vi "UHR-Fleezers Control (host) - 12.7d.vi"() -> ()   [LabVIEW 2012] (continued)
            n1305 = property on="Fish for Tether" class="Bool (strict)"("Val(Sgnl)"=TRUE ("Value (Signaling)")) -> ()  [unwired: 2 in, 2 out]
          }
        }
        n1306 = local write "Cal/Data Acq. Spot"(FALSE ("Cal/Data Acq. Spot")) -> ()
      }
      event "Dump Beads": Value Change {
        n1307 = event-data() -> ()  [unwired: 1 in, 5 out]
        n1308 = flat-sequence {
          tunnel: ["Dump spot flow on?"] -> w1942
          tunnel: [w1953] -> w1943
          tunnel: w1942 -> [w1953]
          tunnel: w1946 -> [w1958]
          tunnel: w1945 -> [w1957]
          tunnel: [w1955] -> w1944
          tunnel: w1943 -> [w1955]
          tunnel: w1944 -> [w1968]
          frame #0 {
            w1947 = FALSE ("Value (Signaling)")
            n1309 = local read "Saving..."() -> (w1949:bool)
            n1310 = local write "Dump Beads"(FALSE ("Dump Beads")) -> ()
            n1311 = property on="Inject Pump 3" class="Bool (strict)"("Val(Sgnl)"=w1947) -> ()  [unwired: 2 in, 2 out]
            n1312 = property on="Inject Pump 1" class="Bool (strict)"("Val(Sgnl)"=w1947) -> ()  [unwired: 2 in, 2 out]
            n1313 = local write "Stop Saving"(w1949) -> ()
          }
          frame #1 {
            w1950 = FALSE ("Fl. Triggered...")
            n1314 = case shown="True" "Dump spot flow on?" {
              frame False {
              }
              frame True {
                n1315 = property on="Sample Channel\nFlow" class="Bool (strict)"("Val(Sgnl)"=TRUE ("Stage Moving")) -> ()  [unwired: 2 in, 2 out]
              }
            }
            n1316 = local write "Fl. Triggered..."(w1950) -> ()
            n1317 = local write "Tether"(w1950) -> ()
            n1318 = property on="Green Laser ON" class="Bool (strict)"("Val(Sgnl)"=w1950) -> ()  [unwired: 2 in, 2 out]
            n1319 = property on="Trap Pos. FB ON" class="Bool (strict)"("Val(Sgnl)"=w1950) -> ()  [unwired: 2 in, 2 out]
            n1320 = property on="Trap Trig. Fl." class="Bool (strict)"("Val(Sgnl)"=w1950) -> ()  [unwired: 2 in, 2 out]
            n1321 = property on="Fl. Triggered..." class="Bool (strict)"("Val(Sgnl)"=w1950) -> ()  [unwired: 2 in, 2 out]
            n1322 = property on="Dip for Protein" class="Bool (strict)"("Val(Sgnl)"=w1950) -> ()  [unwired: 2 in, 2 out]
            n1323 = property on="Pause dwell" class="Bool (strict)"("Val(Sgnl)"=w1950) -> ()  [unwired: 2 in, 2 out]
          }
          frame #2 {
            n1324 = property on="Trap Pos. FB Offset Factor" class="DigNum (strict)"("Val(Sgnl)"=i64 0 ("Value (Signaling)")) -> ()  [unwired: 2 in, 2 out]
          }
          frame #3 {
            n1325 = local read "Saved Stage Positions"() -> (w1959:dbl[][])
            n1326 = local write "Stage Moving"(TRUE ("Stage Moving")) -> ()
            n1327 = Array Subset(array=w1959, index (row)=3 ("index"), length (row)=1 ("length"), index (col)=1 ("index"), length (col)=3 ("length")) -> (w1964:dbl[][])
            n1328 = Reshape Array(w1964, 3 ("dimension size")) -> (w1962:dbl[])
            n1329 = Array To Cluster(array=w1962) -> (cluster=w1961:cluster{"[0]":dbl, "[1]":dbl, "[2]":dbl})
            n1330 = call "Set Stage Position.vi"("Position"=w1961, "error in"=w1957, "VISA resource name in"=w1958) -> ()  [unwired: 3 out]
          }
          frame #4 {
            w1969 = FALSE ("Value (Signaling)")
            n1331 = case shown="True" w1968 {
              frame False {
              }
              frame True {
                n1332 = property on="Sample Channel\nFlow" class="Bool (strict)"("Val(Sgnl)"=FALSE ("Stage Moving")) -> ()  [unwired: 2 in, 2 out]
              }
            }
            n1333 = property on="Trap 1 (ON/OFF)" class="Bool (strict)"("Val(Sgnl)"=w1969) -> ()  [unwired: 2 in, 2 out]
            n1334 = property on="Trap 2 (ON/OFF)" class="Bool (strict)"("Val(Sgnl)"=w1969) -> ()  [unwired: 2 in, 2 out]
            n1335 = call <vilib>:"Beep.vi"() -> ()  [unwired: 3 in, 9 out]
          }
          frame #5 {
            n1336 = property on="Move Cap. 2 (ADig Top)" class="Bool (strict)"("Val(Sgnl)"=TRUE ("Value (Signaling)")) -> ()  [unwired: 2 in, 2 out]
            n1337 = property on="Tab Control" class="TabCtl (strict)"("Val(Sgnl)"=T31."Status" ("Value (Signaling)")) -> ()  [unwired: 2 in, 2 out]
          }
        }
      }
      event "Dip for Protein": Value Change {
        n1338 = event-data() -> ()  [unwired: 1 in, 5 out]
        n1339 = case shown="True" "Dip for Protein" {
          tunnel: w1975 -> [_ w1977]
          tunnel: w1974 -> [_ w1976]
          frame False {
          }
          frame True {
            n1340 = while {
              tunnel: w1977 -> [w1988]
              tunnel: w1976 -> [w1987]
              i -> [w1982]
              stop <- w1984 stop-if-true
              n1341 = Increment(x=w1982) -> (x+1=→"Dip #":i32)
              n1342 = flat-sequence {
                tunnel: w1987 -> [w1999]
                tunnel: w1988 -> [w2000]
                tunnel: [w2000] -> w1992
                tunnel: [w1999] -> w1991
                tunnel: [w1993] -> w1978
                tunnel: [w2005] -> w1986
                tunnel: [w2006] -> w1985
                tunnel: w1992 -> [w2007]
                tunnel: w1991 -> [w2008]
                tunnel: [w2003] -> w1979
                tunnel: w1978 -> [w2003]
                tunnel: [w2016] -> w1990
                tunnel: w1986 -> [w2016]
                tunnel: [w2015] -> w1989
                tunnel: w1985 -> [w2015]
                tunnel: [w2012] -> w1983
                tunnel: [w2011] -> w1980
                tunnel: w1979 -> [w2011]
                tunnel: w1989 -> [w2036]
                tunnel: w1990 -> [w2037]
                tunnel: w1983 -> [w2038]
                tunnel: w1980 -> [w2035]
                tunnel: [w2094] -> w1984
                frame #0 {
                  n1343 = local read "Trap Pos. FB ON"() -> (w1993:bool)
                  n1344 = Compound Arithmetic op=AND("Flow ON\nduring dip?", "FB OFF when \nflow ON", w1993) -> (w1994:bool)
                  n1345 = case shown="True" "Move trap \nbefore dip move?" {
                    frame False {
                    }
                    frame True {
                      n1346 = property on="Trap Delta (MHz)" class="DigNum (strict)"("Val(Sgnl)"="Dipping Delta (MHz)") -> ()  [unwired: 2 in, 2 out]
                    }
                  }
                  n1347 = property on="Green Laser ON" class="Bool (strict)"("Val(Sgnl)"="Green ON\nbefore dip?") -> ()  [unwired: 2 in, 2 out]
                  n1348 = property on="Sample Channel\nFlow" class="Bool (strict)"("Val(Sgnl)"="Flow ON\nduring dip?") -> ()  [unwired: 2 in, 2 out]
                  n1349 = case shown="True" w1994 {
                    frame False {
                    }
                    frame True {
                      n1350 = property on="Trap Pos. FB ON" class="Bool (strict)"("Val(Sgnl)"=FALSE ("Value (Signaling)")) -> ()  [unwired: 2 in, 2 out]
                    }
                  }
                }
                frame #1 {
                  n1351 = local read "Saved Stage Positions"() -> (w2010:dbl[][])
                  n1352 = local write "Cancel dwell"(FALSE ("Cancel dwell")) -> ()
                  n1353 = call "move to saved stage position.vi"("error in"=w2008, "Stage VISA resource name in"=w2007, "Position"="Dip Stage \nPosition", "Saved Stage Positions"=w2010) -> ("VISA resource name out"=w2005:refnum<visa-resource-name>, "error out"=w2006:errorcluster)
                }
                frame #2 {
                  n1354 = node-c288() -> (w2014:T23)  [unwired: 4 in]
                  n1355 = timed-loop {
                    timing: w2014 -> [_]
                    timing-out: [_] -> w2013
                    tunnel: [w2020] -> w2012
                    i -> [w2017]
                    stop <- w2021 stop-if-true
                    n1356 = node-c288() -> ()  [unwired: 1 in, 1 out]
                    n1357 = Greater Or Equal?(x=w2017, y="Dip Duration (s)") -> (x >= y?=w2029:bool)
                    n1358 = local read "Dip for Protein"() -> (w2022:bool)
                    n1359 = local read "Dump Beads"() -> (w2019:bool)
                    n1360 = local read "Cancel dwell"() -> (w2028:bool)
                    n1361 = local read "Pause dwell"() -> (w2025:bool)
                    n1362 = Not(x=w2022) -> (.not. x?=w2027:bool)
                    n1363 = Compound Arithmetic op=OR(w2028, w2029, w2027) -> (w2026:bool)
                    n1364 = Select(t=FALSE, s=w2025, f=w2026) -> (s? t:f=w2023:bool)
                    n1365 = Not(x=w2019) -> (.not. x?=w2018:bool)
                    n1366 = node-c288() -> ()  [unwired: 1 in, 1 out]
                    n1367 = And(x=w2022, y=w2018) -> (x .and. y?=w2020:bool)
                    n1368 = Or(x=w2023, y=w2019) -> (x .or. y?=w2021:bool)
                    "Dip Time (s)" <- w2017
                  }
                  n1369 = node-c288(w2013) -> ()  [unwired: 1 out]
                }
                frame #3 {
                  n1370 = case shown="True" w2038 {
                    tunnel: w2037 -> [_ w2043]
                    tunnel: w2036 -> [_ w2042]
                    tunnel: w2035 -> [_ w2039]
                    frame False {
                    }
                    frame True {
                      n1371 = flat-sequence {
                        tunnel: w2042 -> [w2047]
                        tunnel: w2043 -> [w2048]
                        tunnel: [w2048] -> w2041
                        tunnel: [w2047] -> w2040
                        tunnel: w2039 -> [w2044]
                        tunnel: w2041 -> [w2058]
                        tunnel: w2040 -> [w2057]
                        tunnel: w2039 -> [w2066]
                        frame #0 {
                          n1372 = local read "Sample Channel\nFlow"() -> (w2046:bool)
                          n1373 = case shown="True" w2046 {
                            tunnel: "Flow ON \nduring return\nfrom dip?" -> [w2049 w2052]
                            tunnel: w2044 -> [_ w2051]
                            frame False {
                              n1374 = case shown="True" w2049 {
                                frame False {
                                }
                                frame True {
                                n1375 = property on="Sample Channel\nFlow" class="Bool (strict)"("Val(Sgnl)"=TRUE ("Value (Signaling)")) -> ()  [unwired: 2 in, 2 out]
                                }
                              }
                            }
                            frame True {
                              n1376 = case shown="False" w2052 {
                                tunnel: w2051 -> [w2053 _]
                                frame False {
                                n1377 = property on="Trap Pos. FB ON" class="Bool (strict)"("Val(Sgnl)"=w2053) -> ()  [unwired: 2 in, 2 out]
                                n1378 = property on="Sample Channel\nFlow" class="Bool (strict)"("Val(Sgnl)"=FALSE ("Value (Signaling)")) -> ()  [unwired: 2 in, 2 out]
                                }
                                frame True {
                                }
                              }
                            }
                          }
                        }
                        frame #1 {
                          # "For turning on green laser before stage reaches lower spot"
                          n1379 = case shown="True" "Green ON\nafter start\nreturn?" {
                            frame False {
                            }
                            frame True {
                              n1380 = flat-sequence {
                                frame #0 {
                                n1381 = Multiply(x="Green delay after \nstart return (s)", y=1000.0) -> (x*y=w2063:dbl)
                                n1382 = Wait (ms)(milliseconds to wait=w2063) -> ()  [unwired: 1 out]
                                }
                                frame #1 {
                                n1383 = property on="Green Laser ON" class="Bool (strict)"("Val(Sgnl)"=TRUE ("Value (Signaling)")) -> ()  [unwired: 2 in, 2 out]
                                }
                              }
                            }
                          }
                          n1384 = local read "Saved Stage Positions"() -> (w2061:dbl[][])
                          n1385 = local write "Cancel dwell"(FALSE ("Cancel dwell")) -> ()
                          n1386 = call "move to saved stage position.vi"("error in"=w2057, "Stage VISA resource name in"=w2058, "Position"="Return Stage \nPosition", "Saved Stage Positions"=w2061) -> ("error out"=w2059:errorcluster)  [unwired: 1 out]
                          n1387 = local write "Stage Control Serial Error"(w2059) -> ()
                        }
                        frame #2 {
                          n1388 = property on="Trap Pos. FB ON" class="Bool (strict)"("Val(Sgnl)"=w2066) -> ()  [unwired: 2 in, 2 out]
                          n1389 = case shown="True" "Green ON \nafter return?" {
                            frame False {
                            }
                            frame True {
                              n1390 = property on="Green Laser ON" class="Bool (strict)"("Val(Sgnl)"=TRUE ("Value (Signaling)")) -> ()  [unwired: 2 in, 2 out]
                            }
                          }
                          n1391 = case shown="True" "Move trap after return?" {
                            frame False {
                            }
                            frame True {
                              n1392 = property on="Trap Delta (MHz)" class="DigNum (strict)"("Val(Sgnl)"="Dip Trap Delta 2 (MHz)") -> ()  [unwired: 2 in, 2 out]
                            }
                          }
                          n1393 = case shown="True" "Save data after return?" {
                            frame False {
                            }
                            frame True {
                              n1394 = property on="Start Saving" class="Bool (strict)"("Val(Sgnl)"=TRUE ("Value (Signaling)")) -> ()  [unwired: 2 in, 2 out]
                            }
                          }
                          n1395 = property on="Sample Channel\nFlow" class="Bool (strict)"("Val(Sgnl)"="Flow ON\nduring daq?") -> ()  [unwired: 2 in, 2 out]
                        }
                        frame #3 {
                          n1396 = node-c288() -> (w2075:T23)  [unwired: 4 in]
                          n1397 = timed-loop {
                            timing: w2075 -> [_]
                            timing-out: [_] -> w2074
                            i -> [w2076]
                            stop <- w2078 stop-if-true
                            n1398 = node-c288() -> ()  [unwired: 1 in, 1 out]
                            n1399 = local read "Dump Beads"() -> (w2077:bool)
                            n1400 = Greater Or Equal?(x=w2076, y="Dwell Duration (s)") -> (x >= y?=w2083:bool)
                            n1401 = local read "Dip for Protein"() -> (w2080:bool)
                            n1402 = Not(x=w2080) -> (.not. x?=w2079:bool)
                            n1403 = Compound Arithmetic op=OR(w2083, "Cancel dwell", w2079) -> (w2082:bool)
                            n1404 = node-c288() -> ()  [unwired: 1 in, 1 out]
                            n1405 = Select(t=FALSE, s="Pause dwell", f=w2082) -> (s? t:f=w2085:bool)
                            n1406 = Or(x=w2085, y=w2077) -> (x .or. y?=w2078:bool)
                            "Dwell Time (s)" <- w2076
                          }
                          n1407 = node-c288(w2074) -> ()  [unwired: 1 out]
                        }
                      }
                    }
                  }
                }
                frame #4 {
                  n1408 = local read "Dip for Protein"() -> (w2095:bool)
                  n1409 = local read "Dump Beads"() -> (w2092:bool)
                  n1410 = local write "Cancel dwell"(FALSE ("Cancel dwell")) -> ()
                  n1411 = Not(x=w2095) -> (.not. x?=w2096:bool)
                  n1412 = Not(x="Cont. Repeat Dipping?") -> (.not. x?=w2098:bool)
                  n1413 = Compound Arithmetic op=OR(w2096, w2098, w2092) -> (w2094:bool)
                }
              }
            }
          }
        }
      }
      event "Profile": Value Change {
        n1414 = event-data() -> ()  [unwired: 1 in, 5 out]
        n1415 = flat-sequence {
          tunnel: w2107 -> [w2110]
          tunnel: w2106 -> [w2118]
          tunnel: [w2112] -> w2105
          tunnel: [w2111] -> w2104
          tunnel: [w2109] -> w2102
          tunnel: [w2108] -> w2099
          tunnel: w2105 -> [w2125]
          tunnel: w2104 -> [w2124]
          tunnel: [w2122] -> w2103
          tunnel: w2102 -> [w2123]
          tunnel: [w2121] -> w2101
          tunnel: [w2120] -> w2100
          tunnel: w2099 -> [w2120]
          tunnel: w2103 -> [w2129]
          tunnel: w2101 -> [w2128]
          tunnel: w2100 -> [w2127]
          frame #0 {
            n1416 = call "Read Stage Position.vi"("error in"=w2118, "VISA resource name in"=w2110) -> ("Current Position"=w2108:cluster{dbl, dbl, dbl}, "error out"=w2111:errorcluster, "VISA resource name out"=w2109:refnum<visa-resource-name>)  [unwired: 1 out]
            "Current Position" <- w2108
            n1417 = local write "Stage Control Serial Error"(w2111) -> ()
            n1418 = Unbundle(w2108) -> (w2115:dbl, w2117:dbl, w2113:dbl)
            n1419 = Add(x=w2117, y="Y change (mm)") -> (x+y=w2114:dbl)
            n1420 = Bundle(w2115, w2114, w2113) -> (w2112:cluster{dbl, dbl, dbl})  [unwired: 1 in]
          }
          frame #1 {
            # "move to new position and start saving"
            n1421 = local write "Stage Moving"(TRUE ("Stage Moving")) -> ()
            n1422 = local write "Start Saving"(TRUE ("Start Saving")) -> ()
            n1423 = call "Set Stage Position.vi"("Position"=w2125, "error in"=w2124, "VISA resource name in"=w2123) -> ("error out"=w2121:errorcluster, "VISA resource name out"=w2122:refnum<visa-resource-name>)  [unwired: 1 out]
          }
          frame #2 {
            # "go back to start"
            n1424 = call "Set Stage Position.vi"("Position"=w2127, "error in"=w2128, "VISA resource name in"=w2129) -> ()  [unwired: 3 out]
          }
          frame #3 {
            # "stop saving"
            n1425 = local write "Stop Saving"(TRUE ("Stop Saving")) -> ()
            n1426 = local write "Stage Moving"(FALSE ("Stage Moving")) -> ()
          }
        }
      }
      event "Move to Position 1", "Move to Position 2", "Move to Position 3", "Move to Position 4", "Move to Position 5", "Lower Ch. Cap.": Value Change {
        n1427 = event-data() -> ()  [unwired: 1 in, 5 out]
        n1428 = Or(x="Move to Position 5", y="Lower Ch. Cap.") -> (x .or. y?=w2135:bool)
        n1429 = Build Array("Move to Position 1", "Move to Position 2", "Move to Position 3", "Move to Position 4", w2135) -> (w2138:bool[])
        n1430 = Boolean Array To Number(Boolean array=w2138) -> (number=w2137:u32)
        n1431 = Logarithm Base 2(1:w2137) -> (0:w2136:dbl)
        n1432 = flat-sequence {
          tunnel: w2136 -> [w2147]
          tunnel: w2133 -> [w2145]
          tunnel: w2132 -> [w2144]
          frame #0 {
            n1433 = local read "Saved Stage Positions"() -> (w2155:dbl[][])
            n1434 = Array Subset(array=w2155, index (row)=w2147, length (row)=1 ("length"), index (col)=1 ("index"), length (col)=3 ("length")) -> (w2152:dbl[][])
            n1435 = Reshape Array(w2152, 3 ("dimension size")) -> (w2150:dbl[])
            n1436 = Array To Cluster(array=w2150) -> (cluster=w2149:cluster{"[0]":dbl, "[1]":dbl, "[2]":dbl})
            n1437 = call "Set Stage Position.vi"("Position"=w2149, "error in"=w2144, "VISA resource name in"=w2145) -> ("error out"=w2148:errorcluster)  [unwired: 2 out]
            n1438 = local write "Stage Moving"(TRUE ("Stage Moving")) -> ()
            n1439 = local write "Stage Control Serial Error"(w2148) -> ()
          }
          frame #1 {
            n1440 = local write "Stage Moving"(FALSE ("Stage Moving")) -> ()
            n1441 = call <vilib>:"Beep.vi"() -> ()  [unwired: 3 in, 9 out]
          }
        }
      }
      event "Got ADig bead": Value Change {
        n1442 = event-data() -> ()  [unwired: 1 in, 5 out]
        n1443 = flat-sequence {
          frame #0 {
            n1444 = local read "Cap 1 Samp Flow ON"() -> (w2159:bool)
            n1445 = case shown="True" w2159 {
              frame False {
              }
              frame True {
                n1446 = property on="Sample Channel\nFlow" class="Bool (strict)"("Val(Sgnl)"=TRUE ("Value (Signaling)")) -> ()  [unwired: 2 in, 2 out]
              }
            }
          }
          frame #1 {
            n1447 = property on="Inject Pump 3" class="Bool (strict)"("Val(Sgnl)"=FALSE ("Value (Signaling)")) -> ()  [unwired: 2 in, 2 out]
          }
          frame #2 {
            n1448 = property on="Move Cap. 1 (DNA Bottom)" class="Bool (strict)"("Val(Sgnl)"=TRUE ("Value (Signaling)")) -> ()  [unwired: 2 in, 2 out]
          }
        }
      }
      event "Force FB Data\nScript": Value Change {
        n1449 = event-data() -> ()  [unwired: 1 in, 5 out]
        n1450 = flat-sequence {
          tunnel: w2168 -> [w2172]
          tunnel: w2169 -> [w2173]
          tunnel: [w2173] -> w2164
          tunnel: [w2172] -> w2163
          tunnel: w2164 -> [w2176]
          tunnel: w2163 -> [w2175]
          tunnel: ["Trap Trig Fl."] -> w2165
          tunnel: [w2201] -> w2166
          tunnel: w2165 -> [w2201]
          tunnel: [w2205] -> w2167
          tunnel: w2166 -> [w2205]
          tunnel: w2167 -> [w2207]
          frame #0 {
            n1451 = property on="Trap Delta (MHz)" class="DigNum (strict)"("Val(Sgnl)"="Trap Delta Before Moving") -> ()  [unwired: 2 in, 2 out]
          }
          frame #1 {
            n1452 = local read "Saved Stage Positions"() -> (w2178:dbl[][])
            n1453 = local write "FB Trap Pos Offset"(0.0 ("FB Trap Pos Offset")) -> ()
            n1454 = property on="Trap Pos. FB Offset Factor" class="DigNum (strict)"("Val(Sgnl)"=i64 0 ("Value (Signaling)")) -> ()  [unwired: 2 in, 2 out]
            n1455 = local write "Stage Moving"(TRUE ("Stage Moving")) -> ()
            n1456 = call "move to saved stage position.vi"("error in"=w2175, "Stage VISA resource name in"=w2176, "Position"="Stage Position To Establish FB", "Saved Stage Positions"=w2178) -> ("error out"=w2174:errorcluster)  [unwired: 1 out]
            n1457 = local write "Stage Control Serial Error"(w2174) -> ()
          }
          frame #2 {
            n1458 = call <vilib>:"Beep.vi"() -> ()  [unwired: 3 in, 9 out]
            n1459 = Multiply(x="Wait (s)", y=u32 1000 ("milliseconds to wait")) -> (x*y=w2185:u32)
            n1460 = property on="Trap Delta (MHz)" class="DigNum (strict)"("Val(Sgnl)"="Starting \nTrap Delta (MHz)") -> ()  [unwired: 2 in, 2 out]
            n1461 = local write "Stage Moving"(FALSE ("Stage Moving")) -> ()
            n1462 = Wait (ms)(milliseconds to wait=w2185) -> ()  [unwired: 1 out]
            n1463 = property on="Tab Control 2" class="TabCtl (strict)"("Val(Sgnl)"=T6."Feedback on Trap Position" ("Value (Signaling)")) -> ()  [unwired: 2 in, 2 out]
            n1464 = property on="Tab Control" class="TabCtl (strict)"("Val(Sgnl)"=T32."Trap Control (RF)" ("Value (Signaling)")) -> ()  [unwired: 2 in, 2 out]
          }
          frame #3 {
            n1465 = property on="Set Reading to\nSetpoint" class="Bool (strict)"("Val(Sgnl)"=TRUE ("Value (Signaling)")) -> ()  [unwired: 2 in, 2 out]
            n1466 = Wait (ms)(milliseconds to wait=u32 500) -> ()  [unwired: 1 out]
          }
          frame #4 {
            n1467 = property on="Trap Pos. FB ON" class="Bool (strict)"("Val(Sgnl)"=TRUE ("Value (Signaling)")) -> ()  [unwired: 2 in, 2 out]
            n1468 = Wait (ms)(milliseconds to wait=u32 250) -> ()  [unwired: 1 out]
          }
          frame #5 {
            n1469 = case shown="False" "Trap Trig Fl." {
              frame False {
                n1470 = case shown="True" "Green ON after FB ON?" {
                  selector: "Green ON after FB ON?" -> [_ w2200]
                  frame False {
                  }
                  frame True {
                    n1471 = property on="Green Laser ON" class="Bool (strict)"("Val(Sgnl)"=w2200) -> ()  [unwired: 2 in, 2 out]
                  }
                }
              }
              frame True {
              }
            }
            n1472 = case shown="True" "Remove Action Offset" {
              tunnel: TRUE ("Value (Signaling)") -> [w2197 w2198]
              frame False {
                n1473 = property on="Remove Unwinding Offset" class="Bool (strict)"("Val(Sgnl)"=w2197) -> ()  [unwired: 2 in, 2 out]
              }
              frame True {
                n1474 = property on="Remove Action Offset" class="Bool (strict)"("Val(Sgnl)"=w2198) -> ()  [unwired: 2 in, 2 out]
              }
            }
            n1475 = Wait (ms)(milliseconds to wait=u32 250) -> ()  [unwired: 1 out]
          }
          frame #6 {
            n1476 = property on="Start Saving" class="Bool (strict)"("Val(Sgnl)"=TRUE ("Value (Signaling)")) -> ()  [unwired: 2 in, 2 out]
            n1477 = Wait (ms)(milliseconds to wait=u32 5000) -> ()  [unwired: 1 out]
          }
          frame #7 {
            w2204 = TRUE ("Value (Signaling)")
            n1478 = property on="Rem fb disp offset" class="Bool (strict)"("Val(Sgnl)"=w2204) -> ()  [unwired: 2 in, 2 out]
            n1479 = property on="Remove Offset" class="Bool (strict)"("Val(Sgnl)"=w2204) -> ()  [unwired: 2 in, 2 out]
            n1480 = Wait (ms)(milliseconds to wait=u32 100) -> ()  [unwired: 1 out]
          }
          frame #8 {
            n1481 = case shown="True" w2207 {
              frame False {
              }
              frame True {
                n1482 = local write "Trap Trig. Fl."(TRUE ("Value (Signaling)")) -> ()
              }
            }
          }
          frame #9 {
            n1483 = case shown="True" "Start dipping after?" {
              frame False {
              }
              frame True {
                n1484 = flat-sequence {
                  frame #0 {
                    n1485 = Multiply(x="Delay before dipping (s)", y=1000.0) -> (x*y=w2211:dbl)
                    n1486 = Wait (ms)(milliseconds to wait=w2211) -> ()  [unwired: 1 out]
                  }
                  frame #1 {
                    n1487 = property on="Dip for Protein" class="Bool (strict)"("Val(Sgnl)"=TRUE ("Value (Signaling)")) -> ()  [unwired: 2 in, 2 out]
                    n1488 = local write "Scripts"(T1."Dipping" ("Scripts")) -> ()
                  }
                }
              }
            }
          }
        }
      }
      event "Fixed Traps Data\nScript": Value Change {
        n1489 = event-data() -> ()  [unwired: 1 in, 5 out]
        n1490 = flat-sequence {
          frame #0 {
            n1491 = case shown="True" "Green ON" {
              frame False {
              }
              frame True {
                n1492 = property on="Green Laser ON" class="Bool (strict)"("Val(Sgnl)"=TRUE) -> ()  [unwired: 2 in, 2 out]
              }
            }
            n1493 = local write "Offset (nm)"(0.0 ("Offset (nm)")) -> ()
            n1494 = property on="Sample Channel\nFlow" class="Bool (strict)"("Val(Sgnl)"=FALSE ("Value (Signaling)")) -> ()  [unwired: 2 in, 2 out]
            n1495 = property on="Trap Delta (MHz)" class="DigNum (strict)"("Val(Sgnl)"="Fixed Traps Trap Delta (MHz)") -> ()  [unwired: 2 in, 2 out]
          }
          frame #1 {
            n1496 = Wait (ms)(milliseconds to wait=u32 1000) -> ()  [unwired: 1 out]
          }
          frame #2 {
            n1497 = local write "Start Saving"(TRUE ("Start Saving")) -> ()
          }
          frame #3 {
            n1498 = local read "Bead Sep. Int. Time (s)"() -> (w2222:dbl)
            n1499 = Multiply(x=w2222, y=1000.0) -> (x*y=w2224:dbl)
            n1500 = Wait (ms)(milliseconds to wait=w2224) -> ()  [unwired: 1 out]
          }
          frame #4 {
            n1501 = property on="Remove Offset" class="Bool (strict)"("Val(Sgnl)"=TRUE ("Value (Signaling)")) -> ()  [unwired: 2 in, 2 out]
          }
          frame #5 {
            n1502 = property on="Dip for Protein" class="Bool (strict)"("Val(Sgnl)"="Start dipping after?") -> ()  [unwired: 2 in, 2 out]
          }
        }
      }
      event "Got DNA bead": Value Change {
        n1503 = event-data() -> ()  [unwired: 1 in, 5 out]
        n1504 = flat-sequence {
          frame #0 {
            n1505 = local read "Daq spot flow on"() -> (w2229:bool)
            n1506 = case shown="True" w2229 {
              frame False {
              }
              frame True {
                n1507 = property on="Sample Channel\nFlow" class="Bool (strict)"("Val(Sgnl)"=TRUE ("Value (Signaling)")) -> ()  [unwired: 2 in, 2 out]
              }
            }
            n1508 = property on="Got DNA bead" class="Bool"("Key Focus"=FALSE) -> ()  [unwired: 2 in, 2 out]
          }
          frame #1 {
            n1509 = property on="Inject Pump 1" class="Bool (strict)"("Val(Sgnl)"=FALSE ("Value (Signaling)")) -> ()  [unwired: 2 in, 2 out]
          }
          frame #2 {
            n1510 = property on="Cal/Data Acq. Spot" class="Bool (strict)"("Val(Sgnl)"=TRUE ("Value (Signaling)")) -> ()  [unwired: 2 in, 2 out]
          }
        }
      }
      event "Take Stepping Data": Value Change {
        n1511 = event-data() -> ()  [unwired: 1 in, 5 out]
        n1512 = local read "Save ave N"() -> (w2241:dbl)
        n1513 = flat-sequence {
          tunnel: w2241 -> [w2243]
          tunnel: [w2243] -> w2236
          tunnel: [w2245] -> w2237
          tunnel: w2236 -> [w2245]
          tunnel: [w2247] -> w2238
          tunnel: w2237 -> [w2247]
          tunnel: [w2250] -> w2239
          tunnel: w2238 -> [w2250]
          tunnel: [w2252] -> w2240
          tunnel: w2239 -> [w2252]
          tunnel: [w2254] -> w2234
          tunnel: w2240 -> [w2254]
          tunnel: w2234 -> [w2257]
          tunnel: [w2257] -> w2233
          tunnel: w2233 -> [w2258]
          tunnel: [w2258] -> w2235
          tunnel: w2235 -> [w2264]
          frame #0 {
            n1514 = property on="Save ave N" class="DigNum (strict)"("Val(Sgnl)"="Save ave factor") -> ()  [unwired: 2 in, 2 out]
          }
          frame #1 {
            n1515 = Wait (ms)(milliseconds to wait=u32 100) -> ()  [unwired: 1 out]
          }
          frame #2 {
            n1516 = local read "Offset 2 Start (MHz)"() -> (w2249:dbl)
            n1517 = property on="Saved AOD Raster Scan Parameter Sets" class="Arr (strict)"("Index Values"=u32[] [2]) -> ()  [unwired: 2 in, 2 out]
            n1518 = property on="Trap Delta (MHz)" class="DigNum (strict)"("Val(Sgnl)"=w2249) -> ()  [unwired: 2 in, 2 out]
          }
          frame #3 {
            n1519 = property on="Load parameters" class="Bool (strict)"("Val(Sgnl)"=TRUE ("Value (Signaling)")) -> ()  [unwired: 2 in, 2 out]
          }
          frame #4 {
            n1520 = Wait (ms)(milliseconds to wait=u32 100) -> ()  [unwired: 1 out]
          }
          frame #5 {
            n1521 = property on="Trap Raster Scan" class="Bool (strict)"("Val(Sgnl)"=TRUE ("Value (Signaling)")) -> ()  [unwired: 2 in, 2 out]
          }
          frame #6 {
            n1522 = Wait (ms)(milliseconds to wait=u32 1000) -> ()  [unwired: 1 out]
          }
          frame #7 {
            n1523 = while {
              stop <- w2261 stop-if-true
              n1524 = local read "Raster Scanning..."() -> (w2263:bool)
              n1525 = local read "Saving..."() -> (w2262:bool)
              n1526 = Not(x=w2262) -> (.not. x?=w2259:bool)
              n1527 = Not(x=w2263) -> (.not. x?=w2260:bool)
              n1528 = And(x=w2260, y=w2259) -> (x .and. y?=w2261:bool)
            }
          }
          frame #8 {
            n1529 = property on="Save ave N" class="DigNum (strict)"("Val(Sgnl)"=w2264) -> ()  [unwired: 2 in, 2 out]
          }
        }
      }
      event "Step Size (nm)": Value Change {
        n1530 = event-data() -> ()  [unwired: 1 in, 5 out]
        n1531 = flat-sequence {
          frame #0 {
            n1532 = property on="Saved AOD Raster Scan Parameter Sets" class="Arr (strict)"("Index Values"=u32[] [1]) -> ()  [unwired: 2 in, 2 out]
          }
          frame #1 {
            n1533 = Multiply(x="N Steps", y="Step Size (nm)") -> (x*y=w2266:dbl)
            n1534 = property on="Scan Speed AOD (nm/s) 2" class="DigNum (strict)"("Value"="Step Size (nm)") -> ()  [unwired: 2 in, 2 out]
            n1535 = property on="Step Size AOD (nm) 2" class="DigNum (strict)"("Value"="Step Size (nm)") -> ()  [unwired: 2 in, 2 out]
            n1536 = property on="Scan Range AOD (nm) 2" class="DigNum (strict)"("Value"=w2266) -> ()  [unwired: 2 in, 2 out]
          }
        }
      }
      event "Take Detection Laser\nImage": Value Change {
        n1537 = event-data() -> ()  [unwired: 1 in, 5 out]
        n1538 = flat-sequence {
          tunnel: [w2294] -> w2284
          tunnel: [w2293] -> w2277
          tunnel: [w2292] -> w2269
          tunnel: [w2297] -> w2285
          tunnel: w2284 -> [w2297]
          tunnel: [w2296] -> w2278
          tunnel: w2277 -> [w2296]
          tunnel: [w2295] -> w2270
          tunnel: w2269 -> [w2295]
          tunnel: [w2301] -> w2286
          tunnel: w2285 -> [w2301]
          tunnel: [w2300] -> w2279
          tunnel: w2278 -> [w2300]
          tunnel: [w2299] -> w2271
          tunnel: w2270 -> [w2299]
          tunnel: [w2307] -> w2287
          tunnel: w2286 -> [w2307]
          tunnel: [w2306] -> w2280
          tunnel: w2279 -> [w2306]
          tunnel: [w2305] -> w2272
          tunnel: w2271 -> [w2305]
          tunnel: [w2311] -> w2288
          tunnel: w2287 -> [w2311]
          tunnel: [w2310] -> w2281
          tunnel: w2280 -> [w2310]
          tunnel: [w2309] -> w2273
          tunnel: w2272 -> [w2309]
          tunnel: [w2315] -> w2289
          tunnel: w2288 -> [w2315]
          tunnel: [w2314] -> w2282
          tunnel: w2281 -> [w2314]
          tunnel: [w2313] -> w2274
          tunnel: w2273 -> [w2313]
          tunnel: [w2319] -> w2290
          tunnel: w2289 -> [w2319]
          tunnel: [w2318] -> w2283
          tunnel: w2282 -> [w2318]
          tunnel: [w2317] -> w2275
          tunnel: w2274 -> [w2317]
          tunnel: w2290 -> [w2325]
          tunnel: w2283 -> [w2324]
          tunnel: [w2322] -> w2276
          tunnel: w2275 -> [w2322]
          tunnel: w2276 -> [w2326]
          frame #0 {
            n1539 = local read "Laser interlacing mode"() -> (w2293:enum32{"Laser ON", "Laser OFF", "Interlace"})
            n1540 = local read "Green FB On/Off"() -> (w2292:bool)
            n1541 = local read "Green Laser ON"() -> (w2294:bool)
          }
          frame #1 {
            n1542 = property on="Green FB On/Off" class="Bool (strict)"("Val(Sgnl)"=FALSE ("Value (Signaling)")) -> ()  [unwired: 2 in, 2 out]
          }
          frame #2 {
            n1543 = property on="Green Laser ON" class="Bool (strict)"("Val(Sgnl)"=TRUE ("Value (Signaling)")) -> ()  [unwired: 2 in, 2 out]
            n1544 = property on="Flip Green Filter" class="Bool (strict)"("Val(Sgnl)"=TRUE ("Value (Signaling)")) -> ()  [unwired: 2 in, 2 out]
            n1545 = property on="Laser interlacing mode" class="RadioBtnsControl (strict)"("Val(Sgnl)"=enum32{"Laser ON", "Laser OFF", "Interlace"}."Laser ON" ("Value (Signaling)")) -> ()  [unwired: 2 in, 2 out]
          }
          frame #3 {
            n1546 = Wait (ms)(milliseconds to wait=u32 500) -> ()  [unwired: 1 out]
          }
          frame #4 {
            n1547 = property on="Confocal Image" class="Bool (strict)"("Val(Sgnl)"=TRUE ("Value (Signaling)")) -> ()  [unwired: 2 in, 2 out]
          }
          frame #5 {
            n1548 = Wait (ms)(milliseconds to wait=u32 2000) -> ()  [unwired: 1 out]
          }
          frame #6 {
            n1549 = while {
              stop <- w2320 stop-if-true
              n1550 = local read "Saving..."() -> (w2321:bool)
              n1551 = Not(x=w2321) -> (.not. x?=w2320:bool)
            }
          }
          frame #7 {
            n1552 = property on="Flip Green Filter" class="Bool (strict)"("Val(Sgnl)"=TRUE ("Value (Signaling)")) -> ()  [unwired: 2 in, 2 out]
            n1553 = property on="Green Laser ON" class="Bool (strict)"("Val(Sgnl)"=w2325) -> ()  [unwired: 2 in, 2 out]
            n1554 = property on="Laser interlacing mode" class="RadioBtnsControl (strict)"("Val(Sgnl)"=w2324) -> ()  [unwired: 2 in, 2 out]
          }
          frame #8 {
            n1555 = property on="Green FB On/Off" class="Bool (strict)"("Val(Sgnl)"=w2326) -> ()  [unwired: 2 in, 2 out]
          }
        }
      }
      event "Move in a Circle": Value Change {
        w2327 = dbl[] []
        # "converting distance (d) to angle (a)\na=arcsin(d/2r)"
        # "radius"
        # "radius"
        # "T1 Y"
        # "T1 X"
        n1556 = event-data() -> ()  [unwired: 1 in, 5 out]
        n1557 = local read "BD 1 Frequency 1 (MHz)"() -> (w2335:dbl)
        n1558 = local read "BD 2 Frequency 1 (MHz)"() -> (w2334:dbl)
        n1559 = local read "BD 1 Frequency 2 (MHz)"() -> (w2333:dbl)
        n1560 = local read "BD 2 Frequency 2 (MHz)"() -> (w2332:dbl)
        n1561 = Subtract(x=w2334, y="Center Y Frequency (MHz)") -> (x-y=w2339:dbl)
        n1562 = Absolute Value(x=w2339) -> (abs(x)=w2330:dbl)
        n1563 = flat-sequence {
          tunnel: w2330 -> [w2342]
          tunnel: [w2342] -> w2329
          frame #0 {
            n1564 = local write "Radius (MHz)"(w2342) -> ()
          }
        }
        n1565 = node-c288("Time step (ms)") -> (w2341:T23)  [unwired: 3 in]
        n1566 = timed-loop {
          timing: w2341 -> [_]
          timing-out: [_] -> w2340
          tunnel: w2335 -> [w2425]
          tunnel: w2334 -> [_]
          tunnel: w2333 -> [w2429]
          tunnel: w2332 -> [_]
          tunnel: "Center Y Frequency (MHz)" -> [w2417]
          shift-right: [w2371] -> _
          shift-left: w2327 -> [w2378]
          shift-right: [w2369] -> _
          shift-left: w2327 -> [w2377]
          shift-right: [w2362] -> _
          shift-left: w2327 -> [w2375]
          shift-right: [w2360] -> _
          shift-left: w2327 -> [w2374]
          tunnel: "Move in a Circle" -> [_]
          tunnel: ["Back to start on finish?"] -> w2331
          tunnel: w2329 -> [_]
          tunnel: w2328 -> [w2395]
          tunnel: w2327 -> [w2373]
          i -> [w2390]
          stop <- w2423 stop-if-true
          w2359 = 0 ("index")
          w2380 = 1 ("dimension size")
          # "Trap 2"
          # "Trap 1"
          # "ignore if N = 0"
          # "r"
          # "r"
          # "r"
          # "r"
          # "\"omega*t\""
          # "Trap 2"
          # "Trap separation (radians)"
          # "Trap 1"
          # "Offset (starts\n at bottom of\n the circle)"
          # "\"t\""
          # "omega"
          n1567 = node-c288() -> (w2438:i64)  [unwired: 1 in]
          n1568 = Divide(x=w2438, y=1000) -> (x/y=w2437:dbl)
          n1569 = Divide(x="2D Motion Trap Separation (MHz)", y="Radius (MHz)") -> (x/y=w2405:dbl)
          n1570 = Multiply(x=w2437, y=w2390) -> (x*y=w2409:dbl)
          n1571 = Inverse Sine(1:w2405) -> ()  [unwired: 1 out]
          n1572 = Multiply(x=w2409, y=-1.0) -> (x*y=w2410:dbl)
          n1573 = Multiply(x=6.283185307179586, y="2D Motion Frequency (Hz)") -> (x*y=w2419:dbl)
          n1574 = Select(t=w2409, s="Counterclockwise/Clockwise", f=w2410) -> (s? t:f=w2408:dbl)
          n1575 = Multiply(x=w2419, y=w2408) -> (x*y=w2388:dbl)
          n1576 = Divide(x="Trap 2 phase shift (deg)", y=360.0) -> (x/y=w2396:dbl)
          n1577 = Multiply(x=6.283185307179586, y=w2396) -> (x*y=w2393:dbl)
          n1578 = Add(x=w2388, y=w2393) -> (x+y=w2402:dbl)
          n1579 = Add(x=w2388, y=1.5707963267948966) -> (x+y=w2435:dbl)
          n1580 = Add(x=w2402, y=1.5707963267948966) -> (x+y=w2420:dbl)
          n1581 = Cosine(x=w2435) -> (cos(x)=w2434:dbl)
          n1582 = Sine(x=w2435) -> (sin(x)=w2433:dbl)
          n1583 = Multiply(x=w2434, y="Radius (MHz)") -> (x*y=w2427:dbl)
          n1584 = Cosine(x=w2420) -> (cos(x)=w2432:dbl)
          n1585 = Sine(x=w2420) -> (sin(x)=w2431:dbl)
          n1586 = Multiply(x=w2433, y="Radius (MHz)") -> (x*y=w2426:dbl)
          n1587 = Multiply(x=w2432, y="Radius (MHz)") -> (x*y=w2430:dbl)
          n1588 = Multiply(x=w2431, y="Radius (MHz)") -> (x*y=w2428:dbl)
          n1589 = Add(x=w2427, y=w2425) -> (x+y=w2368:dbl)
          n1590 = Add(x=w2426, y=w2417) -> (x+y=w2366:dbl)
          n1591 = Greater Or Equal?(x=w2390, y="N steps then stop") -> (x >= y?=w2416:bool)
          n1592 = Add(x=w2430, y=w2429) -> (x+y=w2357:dbl)
          n1593 = Add(x=w2428, y=w2417) -> (x+y=w2355:dbl)
          n1594 = Not Equal To 0?(x="N steps then stop") -> (x != 0?=w2412:bool)
          n1595 = And(x=w2416, y=w2412) -> (x .and. y?=w2413:bool)
          n1596 = local read "Trap 1 sum mean"() -> (w2391:dbl)
          n1597 = local read "Stop All"() -> (w2422:bool)
          n1598 = local write "BD 1 Frequency 1 (MHz)"(w2368) -> ()
          n1599 = local write "BD 2 Frequency 1 (MHz)"(w2366) -> ()
          n1600 = local write "BD 1 Frequency 2 (MHz)"(w2357) -> ()
          n1601 = local write "BD 2 Frequency 2 (MHz)"(w2355) -> ()
          n1602 = Select(t=w2390, s="test", f=w2391) -> (s? t:f=→"Waveform Chart":dbl)
          n1603 = Compound Arithmetic op=OR(w2422, "Stop Moving", w2413) -> (w2423:bool)
          n1604 = local read "BD 1 Frequency 3 (MHz)"() -> (w2401:dbl)
          n1605 = local read "BD 2 Frequency 3 (MHz)"() -> (w2400:dbl)
          n1606 = Select(t=w2373, s="Reset graph", f=w2374) -> (s? t:f=w2354:dbl[])
          n1607 = Select(t=w2373, s="Reset graph", f=w2375) -> (s? t:f=w2356:dbl[])
          n1608 = Select(t=w2373, s="Reset graph", f=w2377) -> (s? t:f=w2365:dbl[])
          n1609 = Select(t=w2373, s="Reset graph", f=w2378) -> (s? t:f=w2367:dbl[])
          n1610 = Initialize Array(w2355, w2380) -> (w2381:dbl[])
          n1611 = Initialize Array(w2366, w2380) -> (w2384:dbl[])
          n1612 = Initialize Array(w2357, w2380) -> (w2382:dbl[])
          n1613 = Initialize Array(w2368, w2380) -> (w2385:dbl[])
          n1614 = local read "Y RF Frequency Limits (MHz)"() -> (w2398:T16)
          n1615 = local read "X RF Frequency Limits (MHz)"() -> (w2399:T16)
          n1616 = call "set RF board frequency - interlace.vi"("Board 2 Frequency Limits"=w2398, "Board 1 Frequency Limits"=w2399, "FPGA VI Reference In"=w2395, "Board 2 Frequency 3 (MHz)"=w2400, "Board 1 Frequency 3 (MHz)"=w2401, "Board 2 Frequency 2 (MHz)"=w2355, "Board 2 Frequency 1 (MHz)"=w2366, "Board 1 Frequency 2 (MHz)"=w2357, "Board 1 Frequency 1  (MHz)"=w2368) -> ()  [unwired: 1 in, 2 out]
          n1617 = Bundle(w2382, w2381) -> (w2353:cluster{dbl[], dbl[]})  [unwired: 1 in]
          n1618 = Bundle(w2385, w2384) -> (w2383:cluster{dbl[], dbl[]})  [unwired: 1 in]
          n1619 = Build Array (concatenate)(w2368, w2367) -> (w2372:dbl[])
          n1620 = Build Array (concatenate)(w2366, w2365) -> (w2370:dbl[])
          n1621 = Build Array (concatenate)(w2357, w2356) -> (w2363:dbl[])
          n1622 = Build Array (concatenate)(w2355, w2354) -> (w2361:dbl[])
          n1623 = Bundle(w2372, w2370) -> (w2352:cluster{dbl[], dbl[]})  [unwired: 1 in]
          n1624 = Bundle(w2363, w2361) -> (w2379:cluster{dbl[], dbl[]})  [unwired: 1 in]
          n1625 = Build Array(w2383, w2353, w2352, w2379) -> (→"Trap trajectories":cluster{dbl[], dbl[]}[])
          n1626 = Decrement(x="N steps to plot") -> (x-1=w2358:i32)
          n1627 = Array Subset(array=w2370, index=w2359, length=w2358) -> (w2369:dbl[])
          n1628 = Array Subset(array=w2372, index=w2359, length=w2358) -> (w2371:dbl[])
          n1629 = Array Subset(array=w2363, index=w2359, length=w2358) -> (w2362:dbl[])
          n1630 = Array Subset(array=w2361, index=w2359, length=w2358) -> (w2360:dbl[])
          n1631 = node-c288() -> ()  [unwired: 1 in, 1 out]
        }
        n1632 = node-c288(w2340) -> ()  [unwired: 1 out]
        n1633 = case shown="True" w2331 {
          tunnel: w2335 -> [_ w2346]
          tunnel: w2334 -> [_ w2345]
          tunnel: w2333 -> [_ w2344]
          tunnel: w2332 -> [_ w2343]
          frame False {
          }
          frame True {
            n1634 = flat-sequence {
              tunnel: w2346 -> [w2350]
              tunnel: w2345 -> [w2349]
              tunnel: w2344 -> [w2348]
              tunnel: w2343 -> [w2347]
              frame #0 {
                n1635 = local write "BD 1 Frequency 1 (MHz)"(w2350) -> ()
                n1636 = local write "BD 2 Frequency 1 (MHz)"(w2349) -> ()
                n1637 = local write "BD 1 Frequency 2 (MHz)"(w2348) -> ()
                n1638 = local write "BD 2 Frequency 2 (MHz)"(w2347) -> ()
              }
              frame #1 {
                n1639 = property on="Update all trap values" class="Bool (strict)"("Val(Sgnl)"=TRUE ("Value (Signaling)")) -> ()  [unwired: 2 in, 2 out]
              }
            }
          }
        }
      }
      event "Stop All": Value Change {
        # "Stopping blue laser before shutting off program"
        n1640 = event-data() -> ()  [unwired: 1 in, 5 out]
        n1641 = local read "Delay (ms)"() -> (w2449:i32)
        n1642 = call "serial write macro.vi"("String"="l0", "Delay (ms)"=w2449, "VISA resource name"=w2452) -> ("read buffer"=w2447:string, "error out"=w2448:errorcluster, "VISA resource name out"=w2451:refnum<visa-resource-name>)
        n1643 = local write "read blue buffer"(w2447) -> ()
        n1644 = local write "Blue Error Out"(w2448) -> ()
        n1645 = VISA Close(VISA resource name=w2451) -> ()  [unwired: 1 in, 1 out]
        n1646 = local read "Stop All"() -> (w2453:bool)
      }
    }
    n1647 = node-c288() -> ()  [unwired: 1 in, 1 out]
  }
  n1648 = timed-loop "Oscillate Trap/AOM (fishing, conjugate plane alignment)" {
    tunnel: [w2455] -> w69
    timing: w64 -> [_]
    timing-out: [_] -> w63
    tunnel: w5 -> [w2454]
    stop <- w2455 stop-if-true
    n1649 = node-c288() -> ()  [unwired: 2 out]
    n1650 = event shown="[0] \"Oscillate Set 1\", \"Fish for Tether\": Value Change" {
      selector: _ -> [_ _ _]
      dyn-events: _ -> [_ _ _]
      timeout: _ -> [_ _ _]
      tunnel: [FALSE ("Stop All") _ w3060] -> w2455
      tunnel: w2454 -> [w2458 _ _]
      event "Oscillate Set 1", "Fish for Tether": Value Change {
        n1651 = event-data() -> ()  [unwired: 6 out]
        n1652 = local read "Oscillate Set 1"() -> (w2462:bool)
        n1653 = Or(x=w2462, y="Fish for Tether") -> (x .or. y?=w2460:bool)
        n1654 = case shown="True" w2460 {
          tunnel: "Fish for Tether" -> [_ w2465]
          tunnel: w2458 -> [_ w2463]
          frame False {
          }
          frame True {
            n1655 = case shown="True" w2465 {
              selector: w2465 -> [w2468 w2474]
              tunnel: [w2468 w2474] -> w2464
              frame False {
              }
              frame True {
                n1656 = local write "Scan axis 2"(TRUE) -> ()
                n1657 = local write "Tether"(FALSE ("Tether")) -> ()
                n1658 = local read "Flow ON during cal?"() -> (w2469:bool)
                n1659 = property on="Trap Delta (MHz)" class="DigNum (strict)"("Val(Sgnl)"="Furthest Delta (MHz)") -> ()  [unwired: 2 in, 2 out]
                n1660 = Or(x="Flow ON during \nfishing?", y=w2469) -> (x .or. y?=w2470:bool)
                n1661 = Wait (ms)(milliseconds to wait=u32 500) -> ()  [unwired: 1 out]
                n1662 = property on="Sample Channel\nFlow" class="Bool (strict)"("Val(Sgnl)"=w2470) -> ()  [unwired: 2 in, 2 out]
              }
            }
            n1663 = node-c288() -> (w2467:T23)  [unwired: 1 in, 3 out]
            n1664 = timed-loop "Oscillate AOD" {
              timing: w2467 -> [_]
              timing-out: [_] -> w2466
              tunnel: w2464 -> [w2478]
              tunnel: w2463 -> [w2477]
              i -> [w2486]
              stop <- w2484 stop-if-true
              n1665 = node-c288() -> (w2485:i64)  [unwired: 1 out]
              n1666 = flat-sequence {
                tunnel: w2486 -> [w2513]
                tunnel: w2485 -> [w2512]
                tunnel: w2478 -> [w2496]
                tunnel: [w2496] -> w2483
                tunnel: [w2495] -> w2482
                tunnel: [w2494] -> w2481
                tunnel: [w2491] -> w2479
                tunnel: w2477 -> [w2487]
                tunnel: w2483 -> [w2558]
                tunnel: w2482 -> [w2556]
                tunnel: w2481 -> [w2555]
                tunnel: [w2554] -> w2480
                tunnel: w2479 -> [w2553]
                tunnel: [w2630] -> w2484
                tunnel: w2480 -> [w2629]
                frame #0 {
                  # "w (rad/s)"
                  # "t (s)"
                  n1667 = Divide(x=w2512, y=i64 1000) -> (x/y=w2488:dbl)
                  n1668 = local read "BD 1 Frequency 2 (MHz)"() -> (w2490:dbl)
                  n1669 = Multiply(x="Osc. freq. (Hz)", y=6.283185307179586) -> (x*y=w2510:dbl)
                  n1670 = Multiply(x=w2488, y=w2513) -> (x*y=w2509:dbl)
                  n1671 = Multiply(x=w2510, y=w2509) -> (x*y=w2493:dbl)
                  n1672 = local read "BD 1 Frequency 1 (MHz)"() -> (w2498:dbl)
                  n1673 = case shown="True" w2496 {
                    tunnel: w2493 -> [w2519 w2536]
                    tunnel: w2498 -> [_ w2544]
                    tunnel: w2490 -> [_ w2545]
                    tunnel: [w2516 w2540] -> w2489
                    tunnel: [FALSE w2521] -> w2494
                    tunnel: [0.0 w2532] -> w2491
                    frame False {
                      n1674 = Sine(x=w2519) -> (sin(x)=w2517:dbl)
                      n1675 = Multiply(x=w2517, y="Osc. amp. (MHz)") -> (x*y=w2516:dbl)
                    }
                    frame True {
                      # "trap position goes from 0 to 1 (0 is when it is furthest away, 1 is when closest)\nso we want to test for tether only when farther away, or x < 1"
                      # "quit if taking too long"
                      # "oscillate the trap"
                      # "Test for tether"
                      n1676 = local read "Vec Mean of T1 T2"() -> (w2520:dbl[])
                      "Trigger Signal" <- w2520
                      n1677 = Cosine(x=w2536) -> (cos(x)=w2548:dbl)
                      n1678 = Subtract(x=w2545, y=w2544) -> (x-y=w2543:dbl)
                      n1679 = Decrement(x=w2548) -> (x-1=w2547:dbl)
                      n1680 = Subtract(x=w2543, y="Closest Delta (MHz)") -> (x-y=w2541:dbl)
                      n1681 = Divide(x=w2547, y=-2.0) -> (x/y=w2531:dbl)
                      n1682 = Greater?(x=w2520, y="Stop F (pN)") -> (0:w2538:bool[])
                      n1683 = Multiply(x=w2531, y=w2541) -> (x*y=w2540:dbl)
                      n1684 = Less?(x=w2531, y="Fish mask thresh") -> (x < y?=w2530:bool)
                      n1685 = Boolean To (0,1)(Boolean=w2530) -> (0, 1=w2528:i16)
                      n1686 = Multiply(x=w2528, y=w2520) -> (x*y=w2527:dbl[])
                      n1687 = Divide(x=w2536, y=6.283185307179586) -> (x/y=w2535:dbl)
                      n1688 = Round Toward +Infinity(x=w2535) -> (ceil(x): smallest int >= x=w2532:dbl)
                      "Attempts" <- w2532
                      n1689 = Greater?(x=w2527, y="Stop F (pN) (mask)") -> (0:w2525:bool[])
                      n1690 = Or Array Elements(Boolean array=w2538) -> (logical OR=w2523:bool)
                      n1691 = Or Array Elements(Boolean array=w2525) -> (logical OR=w2522:bool)
                      n1692 = Greater?(x=w2532, y="Attempt Limit") -> (0:w2534:bool)
                      n1693 = case shown="True" w2534 {
                        frame False {
                        }
                        frame True {
                          n1694 = local write "Fish for Tether"(FALSE ("Fish for Tether")) -> ()
                          n1695 = call <vilib>:"Beep.vi"() -> ()  [unwired: 3 in, 9 out]
                          n1696 = local read "Messages"() -> (w2550:string)
                          n1697 = call "Update messages.vi"("Message to add"="Tether fishing timeout." ("Messages"), "Old message string"=w2550) -> ("New message string"=→"Messages":string)
                        }
                      }
                      n1698 = Select(t=w2523, s="Normal (on) or masked test (off)", f=w2522) -> (s? t:f=w2521:bool)